vi "run_pharmaBotExp_v0.015.vi"(0 "data in":T12={"daq_ao 1"="Dev1/ao0", "daq_ai 1"="Dev1/ai0", "experiment day folder"=path "C:/multiBot/data/debug/testing", "Multiclamp init error"=0, "Multiclamp Handle Out"=10225184, "sampling rate (Hz)"=20000, "trial name"="t1"}, 1 "auto run?":bool=TRUE, 3 "which manipulator":T13(ring), 4 "HEK/slice options":enum16{"slice", "HEK"}(ring), 5 "error in":errorcluster, 6 "Validate after Experiment":bool, 7 "common cluster":T9, 11 "individual controls in":T8, 13 "images":T3={"slice image"="remote image 000000001461186C", "pipette template"="remote image 000000001461152C", "found pipette"=refnum, "pipette mask for cell tracker"=refnum, "cell images ref"=refnum}) -> (10 "Cell Looks Good?":bool=TRUE, 12 "ValidationOutputCluster":T5(array[cluster]), 14 "ValidationResults":waveform(dbl)[][](array[waveform]), 15 "ValidationPos1":T6(array[ring]), 16 "Exp. Terminated":bool, 17 "ValidationPos2":T6(array[ring]), 18 "ValidationWaveform":waveform(dbl)[](array[waveform]), 19 "error out":errorcluster)   [LabVIEW 2015] (continued)
  in  "Voltage Pulse K":T25={"Which Position to use for Experiment"=enum."Jumper Safe Position", "Duration (s)"=1.0, "Delay (s)"=0.2, "Pulse 2 (s)"=0.4, "Pulse 1 (mV)"=-80.0, "Replicates"=1.0, "Pulse 1 (s)"=0.2, "Pulse 2 (mV)"=-80.0, "Vholding (mV)"=-60.0, "Valve 1 Position"=2, "Valve 2 Position"=2, "Valve 3 Position"=2, "valve 1 used now?"=TRUE, "valve 2 used now?"=FALSE, "valve 3 used now? "=FALSE, "Maintain Final Voltage until end?"=TRUE, "delta Pulse 1 (mV)"=0.0, "delta Pulse 2 (mV)"=5.0, "Sweeps"=24.0, "Final Pulse 1 (mV)"=0.0, "Final Pulse 2 (mV)"=0.0, "protocol Preview"=[]} {"Final Pulse 2 (mV)" step=0.1; "Final Pulse 1 (mV)" step=0.1; "Sweeps" min=1.0 step=1.0; "delta Pulse 2 (mV)" step=0.1; "delta Pulse 1 (mV)" step=0.1; "Valve 3 Position" min=1 max=8; "Valve 2 Position" min=1 max=8; "Valve 1 Position" min=1 max=8; "Vholding (mV)" step=0.1; "Pulse 2 (mV)" step=0.1; "Pulse 1 (s)" min=0.0 step=0.1; "Replicates" min=1.0 step=1.0; "Pulse 1 (mV)" step=0.1; "Pulse 2 (s)" min=0.0 step=0.1; "Delay (s)" min=0.0 step=0.1; "Duration (s)" min=0.0 step=0.1}
  in  "Jump Train K":T26={"Which Position to use for Experiment"=enum."Jumper Safe Position", "Start Position (N)"="", "Jump Position (m)"="", "Duration (s)"=20.0, "Delay (s)"=1.0, "Pulse Width (s)"=1.0, "Valve 1 Position"=1, "Valve 2 Position"=1, "Replicates"=1.0, "Pulse Period (s)"=2.0, "Vholding (mV)"=-60.0, "Number of Pulses"=5.0, "valve 1 used now?"=TRUE, "valve 2 used now?"=FALSE, "valve 3 used now? "=FALSE, "Valve 3 Position"=1, "protocol Preview"=[]} {"Valve 3 Position" min=1 max=8; "Number of Pulses" min=0.0 step=1.0; "Vholding (mV)" step=0.1; "Pulse Period (s)" min=0.0 step=0.1; "Replicates" min=1.0 step=1.0; "Valve 2 Position" min=1 max=8; "Valve 1 Position" min=1 max=8; "Pulse Width (s)" min=0.0 step=0.1; "Delay (s)" min=0.0 step=0.1; "Duration (s)" min=0.0 step=0.1}
  in  "Paired Pulse K":T27={"Which Position to use for Experiment"=enum."Jumper Safe Position", "Start Position (N)"="", "Jump Position (m)"="", "Duration (s)"=10.0, "Delay (s)"=1.0, "Pulse Width (s)"=1.0, "Replicates"=1.0, "Pulse Delay (s)"=1.0, "Pulse Delta Delay (s)"=0.5, "Vholding (mV)"=-60.0, "Valve 1 Position"=1, "Valve 2 Position"=1, "valve 1 used now?"=TRUE, "valve 2 used now?"=FALSE, "valve 3 used now? "=FALSE, "Valve 3 Position"=1, "protocol Preview"=[]} {"Valve 3 Position" min=1 max=8; "Valve 2 Position" min=1 max=8; "Valve 1 Position" min=1 max=8; "Vholding (mV)" step=0.1; "Pulse Delta Delay (s)" min=0.0 step=0.1; "Pulse Delay (s)" min=0.0 step=0.1; "Replicates" min=1.0 step=1.0; "Pulse Width (s)" min=0.0 step=0.1; "Delay (s)" min=0.0 step=0.1; "Duration (s)" min=0.0 step=0.1}
  in  "Single Manip Jump K":T28={"Start Position (N)"=enum."Jumper Position B", "Duration (s)"=8.0, "Delay (s)"=0.5, "Pulse Width (s)"=1.0, "Valve 1 Position"=2, "Valve 2 Position"=2, "Replicates"=10.0, "Jump Position (m)"=enum."Jumper Position A", "Vholding (mV)"=-60.0, "Valve 3 Position"=2, "valve 1 used now?"=TRUE, "valve 2 used now?"=FALSE, "valve 3 used now? "=FALSE, "protocol Preview"=[]} {"Valve 3 Position" min=1 max=8; "Vholding (mV)" step=0.1; "Replicates" min=1.0 step=1.0; "Valve 2 Position" min=1 max=8; "Valve 1 Position" min=1 max=8; "Pulse Width (s)" min=0.0 step=0.1; "Delay (s)" min=0.0 step=0.1; "Duration (s)" min=0.0 step=0.1}
  in  "Gap Free K":T29={"Which Position to use for Experiment"=enum."Jumper Position B", "Duration (s)"=10.0, "Valve 1 Position"=2, "Valve 2 Position"=2, "Replicates"=5.0, "Vholding (mV)"=-60.0, "Valve 3 Position"=2, "valve 1 used now?"=TRUE, "valve 2 used now?"=FALSE, "valve 3 used now? "=FALSE, "Record During Solution Change?"=FALSE} {"Valve 3 Position" min=1 max=8; "Vholding (mV)" step=0.1; "Replicates" min=1.0 step=1.0; "Valve 2 Position" min=1 max=8; "Valve 1 Position" min=1 max=8; "Duration (s)" min=0.0 step=0.1}
  in  "Multi Manip Jump K":T30={"Start Position (N)"=enum."Jumper Position C", "Duration (s)"=20.0, "Delay (s)"=2.0, "Valve 1 Position"=2, "Valve 2 Position"=2, "Replicates"=5.0, "Vholding (mV)"=-60.0, "Valve 3 Position"=2, "valve 1 used now?"=TRUE, "valve 2 used now?"=FALSE, "valve 3 used now? "=FALSE, "Jump Position Array"=[enum."Jumper Position B", enum."Jumper Position A", enum."Jumper Position B", enum."Jumper Position C"], "Position Dwell Time (s)"=[2.0, 4.0, 4.0, 4.0], "protocol Preview"=[]} {"Position Dwell Time (s)" min=0.0 step=0.1; "Vholding (mV)" step=0.1; "Replicates" min=1.0 step=1.0; "Valve 2 Position" min=1 max=8; "Delay (s)" min=0.0 step=0.1; "Duration (s)" min=0.0 step=0.1}
  in  "Current Pulse K":T31={"Which Position to use for Experiment"=enum."Jumper Safe Position", "Duration (s)"=1.0, "Delay (s)"=0.2, "Pulse 2 (s)"=0.4, "Pulse 1 (pA)"=-400.0, "Replicates"=1.0, "Pulse 1 (s)"=0.6, "Pulse 2 (pA)"=-80.0, "Iholding (pA)"=0.0, "Valve 1 Position"=2, "Valve 2 Position"=2, "Valve 3 Position"=2, "valve 1 used now?"=TRUE, "valve 2 used now?"=FALSE, "valve 3 used now? "=FALSE, "Maintain Final Voltage until end?"=FALSE, "delta Pulse 1 (pA)"=50.0, "delta Pulse 2 (pA)"=5.0, "Sweeps"=24.0, "Final Pulse 1 (pA)"=0.0, "Final Pulse 2 (pA)"=0.0, "protocol Preview"=[]} {"Final Pulse 2 (pA)" step=0.1; "Final Pulse 1 (pA)" step=0.1; "Sweeps" min=1.0 step=1.0; "delta Pulse 2 (pA)" step=0.1; "delta Pulse 1 (pA)" step=0.1; "Valve 3 Position" min=1 max=8; "Valve 2 Position" min=1 max=8; "Valve 1 Position" min=1 max=8; "Iholding (pA)" step=0.1; "Pulse 2 (pA)" step=0.1; "Pulse 1 (s)" min=0.0 step=0.1; "Replicates" min=1.0 step=1.0; "Pulse 1 (pA)" step=0.1; "Pulse 2 (s)" min=0.0 step=0.1; "Delay (s)" min=0.0 step=0.1; "Duration (s)" min=0.0 step=0.1}
  in  "Current Ramp K":T32={"Which Position to use for Experiment"=enum."Jumper Safe Position", "Duration (s)"=10.0, "Delay (s)"=1.0, "Ramp Slope (pA/s)"=0.0, "Current Start (pA)"=-200.0, "Replicates"=1.0, "Current End (pA)"=500.0, "Ramp Duration (s)"=5.0, "Iholding (pA)"=0.0, "Valve 1 Position"=2, "Valve 2 Position"=2, "Valve 3 Position"=2, "valve 1 used now?"=TRUE, "valve 2 used now?"=FALSE, "valve 3 used now? "=FALSE, "Maintain Final Voltage until end?"=FALSE, "protocol Preview"=[]} {"Valve 3 Position" min=1 max=8; "Valve 2 Position" min=1 max=8; "Valve 1 Position" min=1 max=8; "Ramp Duration (s)" min=0.0 step=0.1; "Current End (pA)" step=0.1; "Replicates" min=1.0 step=1.0; "Current Start (pA)" step=0.1; "Ramp Slope (pA/s)" step=0.1; "Delay (s)" min=0.0 step=0.1; "Duration (s)" min=0.0 step=0.1}
  in  "Gap Free Iclamp K":T33={"Which Position to use for Experiment"=enum."Don't Move", "Duration (s)"=10.0, "Valve 1 Position"=2, "Valve 2 Position"=2, "Replicates"=5.0, "Iholding (pA)"=200.0, "Valve 3 Position"=2, "valve 1 used now?"=TRUE, "valve 2 used now?"=FALSE, "valve 3 used now? "=FALSE, "Record During Solution Change?"=FALSE} {"Valve 3 Position" min=1 max=8; "Iholding (pA)" step=0.1; "Replicates" min=1.0 step=1.0; "Valve 2 Position" min=1 max=8; "Valve 1 Position" min=1 max=8; "Duration (s)" min=0.0 step=0.1}
  in  "PhaseL Experiment Option":string(combo)="Single Manip Jump"
  in  "Experiment Selection L":T20(tab)=enum."Paired Pulse"
  in  "Single Jump L":T21={"Which Position to use for Experiment"=enum."Jumper Position B-A", "Start Position (N)"="Jumper Posistion B", "Jump Position (m)"="Jumper Posistion A", "Duration (s)"=5.0, "Delay (s)"=1.0, "Pulse Width (s)"=1.0, "Valve 1 Position"=2, "Valve 2 Position"=2, "Replicates"=10.0, "Vholding (mV)"=-60.0, "Valve 3 Position"=2, "valve 1 used now?"=TRUE, "valve 2 used now?"=FALSE, "valve 3 used now? "=FALSE, "protocol Preview"=[]} {"Valve 3 Position" min=1 max=8; "Vholding (mV)" step=0.1; "Replicates" min=1.0 step=1.0; "Valve 2 Position" min=1 max=8; "Valve 1 Position" min=1 max=8; "Pulse Width (s)" min=0.0 step=0.1; "Delay (s)" min=0.0 step=0.1; "Duration (s)" min=0.0 step=0.1}
  in  "Solution Change L":T22={"Which Position to use for Experiment"=enum."Jumper Safe Position", "Duration (s)"=60.0, "Delay (s)"=1.0, "Pulse Width (s)"=30.0, "Which Valve to Change?"=1, "Valve Jump Position"=3, "Replicates"=1.0, "Vholding (mV)"=-70.0, "valve 1 used now?"=TRUE, "valve 2 used now?"=FALSE, "valve 3 used now? "=FALSE, "Valve 1 Position"=2, "Valve 2 Position"=2, "Valve 3 Position"=2, "protocol Preview"=[]} {"Valve 3 Position" min=1 max=8; "Valve 2 Position" min=1 max=8; "Valve 1 Position" min=1 max=8; "Vholding (mV)" step=0.1; "Replicates" min=1.0 step=1.0; "Valve Jump Position" min=1 max=8 step=1; "Which Valve to Change?" min=1 max=8 step=1; "Pulse Width (s)" min=0.0 step=0.1; "Delay (s)" min=0.0 step=0.1; "Duration (s)" min=0.0 step=0.1}
  in  "Voltage Step L":T23={"Which Position to use for Experiment"=enum."Jumper Safe Position", "Duration (s)"=10.0, "Delay (s)"=1.0, "Step Width (s)"=0.1, "Voltage Start (mV)"=-60.0, "Voltage Step (mV)"=0.0, "Replicates"=1.0, "Voltage End (mV)"=40.0, "Number of Step"=20.0, "Vholding (mV)"=-60.0, "Valve 1 Position"=2, "Valve 2 Position"=2, "Valve 3 Position"=2, "valve 1 used now?"=TRUE, "valve 2 used now?"=FALSE, "valve 3 used now? "=FALSE, "Total Step Time (s)"=0.0, "Maintain Final Voltage until end?"=TRUE, "protocol Preview"=[]} {"Total Step Time (s)" min=0.0 step=0.1; "Valve 3 Position" min=1 max=8; "Valve 2 Position" min=1 max=8; "Valve 1 Position" min=1 max=8; "Vholding (mV)" step=0.1; "Number of Step" min=0.0 step=1.0; "Voltage End (mV)" step=0.1; "Replicates" min=1.0 step=1.0; "Voltage Step (mV)" step=0.1; "Voltage Start (mV)" step=0.1; "Step Width (s)" step=0.1; "Delay (s)" min=0.0 step=0.1; "Duration (s)" min=0.0 step=0.1}
  in  "Voltage Ramp L":T24={"Which Position to use for Experiment"=enum."Jumper Safe Position", "Duration (s)"=10.0, "Delay (s)"=1.0, "Ramp Slope (mV/s)"=0.0, "Voltage Start (mV)"=-60.0, "Replicates"=1.0, "Voltage End (mV)"=40.0, "Ramp Duration (s)"=5.0, "Vholding (mV)"=-60.0, "Valve 1 Position"=2, "Valve 2 Position"=2, "Valve 3 Position"=2, "valve 1 used now?"=TRUE, "valve 2 used now?"=FALSE, "valve 3 used now? "=FALSE, "Maintain Final Voltage until end?"=TRUE, "protocol Preview"=[]} {"Valve 3 Position" min=1 max=8; "Valve 2 Position" min=1 max=8; "Valve 1 Position" min=1 max=8; "Ramp Duration (s)" min=0.0 step=0.1; "Voltage End (mV)" step=0.1; "Replicates" min=1.0 step=1.0; "Voltage Start (mV)" step=0.1; "Ramp Slope (mV/s)" step=0.1; "Delay (s)" min=0.0 step=0.1; "Duration (s)" min=0.0 step=0.1}
  in  "Voltage Pulse L":T25={"Which Position to use for Experiment"=enum."Jumper Safe Position", "Duration (s)"=1.0, "Delay (s)"=0.2, "Pulse 2 (s)"=0.4, "Pulse 1 (mV)"=-80.0, "Replicates"=1.0, "Pulse 1 (s)"=0.2, "Pulse 2 (mV)"=-80.0, "Vholding (mV)"=-60.0, "Valve 1 Position"=2, "Valve 2 Position"=2, "Valve 3 Position"=2, "valve 1 used now?"=TRUE, "valve 2 used now?"=FALSE, "valve 3 used now? "=FALSE, "Maintain Final Voltage until end?"=TRUE, "delta Pulse 1 (mV)"=0.0, "delta Pulse 2 (mV)"=5.0, "Sweeps"=24.0, "Final Pulse 1 (mV)"=0.0, "Final Pulse 2 (mV)"=0.0, "protocol Preview"=[]} {"Final Pulse 2 (mV)" step=0.1; "Final Pulse 1 (mV)" step=0.1; "Sweeps" min=1.0 step=1.0; "delta Pulse 2 (mV)" step=0.1; "delta Pulse 1 (mV)" step=0.1; "Valve 3 Position" min=1 max=8; "Valve 2 Position" min=1 max=8; "Valve 1 Position" min=1 max=8; "Vholding (mV)" step=0.1; "Pulse 2 (mV)" step=0.1; "Pulse 1 (s)" min=0.0 step=0.1; "Replicates" min=1.0 step=1.0; "Pulse 1 (mV)" step=0.1; "Pulse 2 (s)" min=0.0 step=0.1; "Delay (s)" min=0.0 step=0.1; "Duration (s)" min=0.0 step=0.1}
  in  "Jump Train L":T26={"Which Position to use for Experiment"=enum."Jumper Safe Position", "Start Position (N)"="", "Jump Position (m)"="", "Duration (s)"=20.0, "Delay (s)"=1.0, "Pulse Width (s)"=1.0, "Valve 1 Position"=1, "Valve 2 Position"=1, "Replicates"=1.0, "Pulse Period (s)"=2.0, "Vholding (mV)"=-60.0, "Number of Pulses"=5.0, "valve 1 used now?"=TRUE, "valve 2 used now?"=FALSE, "valve 3 used now? "=FALSE, "Valve 3 Position"=1, "protocol Preview"=[]} {"Valve 3 Position" min=1 max=8; "Number of Pulses" min=0.0 step=1.0; "Vholding (mV)" step=0.1; "Pulse Period (s)" min=0.0 step=0.1; "Replicates" min=1.0 step=1.0; "Valve 2 Position" min=1 max=8; "Valve 1 Position" min=1 max=8; "Pulse Width (s)" min=0.0 step=0.1; "Delay (s)" min=0.0 step=0.1; "Duration (s)" min=0.0 step=0.1}
  in  "Paired Pulse L":T27={"Which Position to use for Experiment"=enum."Jumper Safe Position", "Start Position (N)"="", "Jump Position (m)"="", "Duration (s)"=10.0, "Delay (s)"=1.0, "Pulse Width (s)"=1.0, "Replicates"=1.0, "Pulse Delay (s)"=1.0, "Pulse Delta Delay (s)"=0.5, "Vholding (mV)"=-60.0, "Valve 1 Position"=1, "Valve 2 Position"=1, "valve 1 used now?"=TRUE, "valve 2 used now?"=FALSE, "valve 3 used now? "=FALSE, "Valve 3 Position"=1, "protocol Preview"=[]} {"Valve 3 Position" min=1 max=8; "Valve 2 Position" min=1 max=8; "Valve 1 Position" min=1 max=8; "Vholding (mV)" step=0.1; "Pulse Delta Delay (s)" min=0.0 step=0.1; "Pulse Delay (s)" min=0.0 step=0.1; "Replicates" min=1.0 step=1.0; "Pulse Width (s)" min=0.0 step=0.1; "Delay (s)" min=0.0 step=0.1; "Duration (s)" min=0.0 step=0.1}
  in  "Single Manip Jump L":T28={"Start Position (N)"=enum."Jumper Position B", "Duration (s)"=8.0, "Delay (s)"=0.5, "Pulse Width (s)"=1.0, "Valve 1 Position"=2, "Valve 2 Position"=2, "Replicates"=10.0, "Jump Position (m)"=enum."Jumper Position A", "Vholding (mV)"=-60.0, "Valve 3 Position"=2, "valve 1 used now?"=TRUE, "valve 2 used now?"=FALSE, "valve 3 used now? "=FALSE, "protocol Preview"=[]} {"Valve 3 Position" min=1 max=8; "Vholding (mV)" step=0.1; "Replicates" min=1.0 step=1.0; "Valve 2 Position" min=1 max=8; "Valve 1 Position" min=1 max=8; "Pulse Width (s)" min=0.0 step=0.1; "Delay (s)" min=0.0 step=0.1; "Duration (s)" min=0.0 step=0.1}
  in  "Gap Free L":T29={"Which Position to use for Experiment"=enum."Jumper Position B", "Duration (s)"=10.0, "Valve 1 Position"=2, "Valve 2 Position"=2, "Replicates"=5.0, "Vholding (mV)"=-60.0, "Valve 3 Position"=2, "valve 1 used now?"=TRUE, "valve 2 used now?"=FALSE, "valve 3 used now? "=FALSE, "Record During Solution Change?"=FALSE} {"Valve 3 Position" min=1 max=8; "Vholding (mV)" step=0.1; "Replicates" min=1.0 step=1.0; "Valve 2 Position" min=1 max=8; "Valve 1 Position" min=1 max=8; "Duration (s)" min=0.0 step=0.1}
  in  "Multi Manip Jump L":T30={"Start Position (N)"=enum."Jumper Position C", "Duration (s)"=20.0, "Delay (s)"=2.0, "Valve 1 Position"=2, "Valve 2 Position"=2, "Replicates"=5.0, "Vholding (mV)"=-60.0, "Valve 3 Position"=2, "valve 1 used now?"=TRUE, "valve 2 used now?"=FALSE, "valve 3 used now? "=FALSE, "Jump Position Array"=[enum."Jumper Position B", enum."Jumper Position A", enum."Jumper Position B", enum."Jumper Position C"], "Position Dwell Time (s)"=[2.0, 4.0, 4.0, 4.0], "protocol Preview"=[]} {"Position Dwell Time (s)" min=0.0 step=0.1; "Vholding (mV)" step=0.1; "Replicates" min=1.0 step=1.0; "Valve 2 Position" min=1 max=8; "Delay (s)" min=0.0 step=0.1; "Duration (s)" min=0.0 step=0.1}
  in  "Current Pulse L":T31={"Which Position to use for Experiment"=enum."Jumper Safe Position", "Duration (s)"=1.0, "Delay (s)"=0.2, "Pulse 2 (s)"=0.4, "Pulse 1 (pA)"=-400.0, "Replicates"=1.0, "Pulse 1 (s)"=0.6, "Pulse 2 (pA)"=-80.0, "Iholding (pA)"=0.0, "Valve 1 Position"=2, "Valve 2 Position"=2, "Valve 3 Position"=2, "valve 1 used now?"=TRUE, "valve 2 used now?"=FALSE, "valve 3 used now? "=FALSE, "Maintain Final Voltage until end?"=FALSE, "delta Pulse 1 (pA)"=50.0, "delta Pulse 2 (pA)"=5.0, "Sweeps"=24.0, "Final Pulse 1 (pA)"=0.0, "Final Pulse 2 (pA)"=0.0, "protocol Preview"=[]} {"Final Pulse 2 (pA)" step=0.1; "Final Pulse 1 (pA)" step=0.1; "Sweeps" min=1.0 step=1.0; "delta Pulse 2 (pA)" step=0.1; "delta Pulse 1 (pA)" step=0.1; "Valve 3 Position" min=1 max=8; "Valve 2 Position" min=1 max=8; "Valve 1 Position" min=1 max=8; "Iholding (pA)" step=0.1; "Pulse 2 (pA)" step=0.1; "Pulse 1 (s)" min=0.0 step=0.1; "Replicates" min=1.0 step=1.0; "Pulse 1 (pA)" step=0.1; "Pulse 2 (s)" min=0.0 step=0.1; "Delay (s)" min=0.0 step=0.1; "Duration (s)" min=0.0 step=0.1}
  in  "Current Ramp L":T32={"Which Position to use for Experiment"=enum."Jumper Safe Position", "Duration (s)"=10.0, "Delay (s)"=1.0, "Ramp Slope (pA/s)"=0.0, "Current Start (pA)"=-200.0, "Replicates"=1.0, "Current End (pA)"=500.0, "Ramp Duration (s)"=5.0, "Iholding (pA)"=0.0, "Valve 1 Position"=2, "Valve 2 Position"=2, "Valve 3 Position"=2, "valve 1 used now?"=TRUE, "valve 2 used now?"=FALSE, "valve 3 used now? "=FALSE, "Maintain Final Voltage until end?"=FALSE, "protocol Preview"=[]} {"Valve 3 Position" min=1 max=8; "Valve 2 Position" min=1 max=8; "Valve 1 Position" min=1 max=8; "Ramp Duration (s)" min=0.0 step=0.1; "Current End (pA)" step=0.1; "Replicates" min=1.0 step=1.0; "Current Start (pA)" step=0.1; "Ramp Slope (pA/s)" step=0.1; "Delay (s)" min=0.0 step=0.1; "Duration (s)" min=0.0 step=0.1}
  in  "Gap Free Iclamp L":T33={"Which Position to use for Experiment"=enum."Don't Move", "Duration (s)"=10.0, "Valve 1 Position"=2, "Valve 2 Position"=2, "Replicates"=5.0, "Iholding (pA)"=200.0, "Valve 3 Position"=2, "valve 1 used now?"=TRUE, "valve 2 used now?"=FALSE, "valve 3 used now? "=FALSE, "Record During Solution Change?"=FALSE} {"Valve 3 Position" min=1 max=8; "Iholding (pA)" step=0.1; "Replicates" min=1.0 step=1.0; "Valve 2 Position" min=1 max=8; "Valve 1 Position" min=1 max=8; "Duration (s)" min=0.0 step=0.1}
  in  "ending set":enum32{"Iprot", "Vprot", "Imemtest", "Vmemtest"}(tab)
  in  "holding memtest":bool=TRUE
  in  "holding set":enum32{"VClamp", "IClamp"}(tab)
  out "holding vmemtest cmd":waveform(dbl)(graph)
  in  "holding Vclamp memtest":T17={"Samples to Read"=2000, "Rate (Hz)"=20000.0, "Amplitude (mV/pA)"=10.0, "Offset (mV/pA)"=0.0, "Frequency (Hz)"=10.0, "duty cycle (%)"=50.0, "phase"=-90.0} {"phase" format="%.2p"; "duty cycle (%)" format="%0.2f"}
  out "holding imemtest cmd":waveform(dbl)(graph)
  in  "holding Iclamp memtest":T17={"Samples to Read"=2000, "Rate (Hz)"=20000.0, "Amplitude (mV/pA)"=-50.0, "Offset (mV/pA)"=0.0, "Frequency (Hz)"=10.0, "duty cycle (%)"=50.0, "phase"=0.0} {"phase" format="%.2p"; "duty cycle (%)" format="%0.2f"}
  # "(will skip all subsequent Phases)"
  # "Checks Twitter for user Control\npharmaBotEmory\nga12345"
  # "IClamp step protocol"
  # "x"
  # "VClamp step protocol"
  # "x"
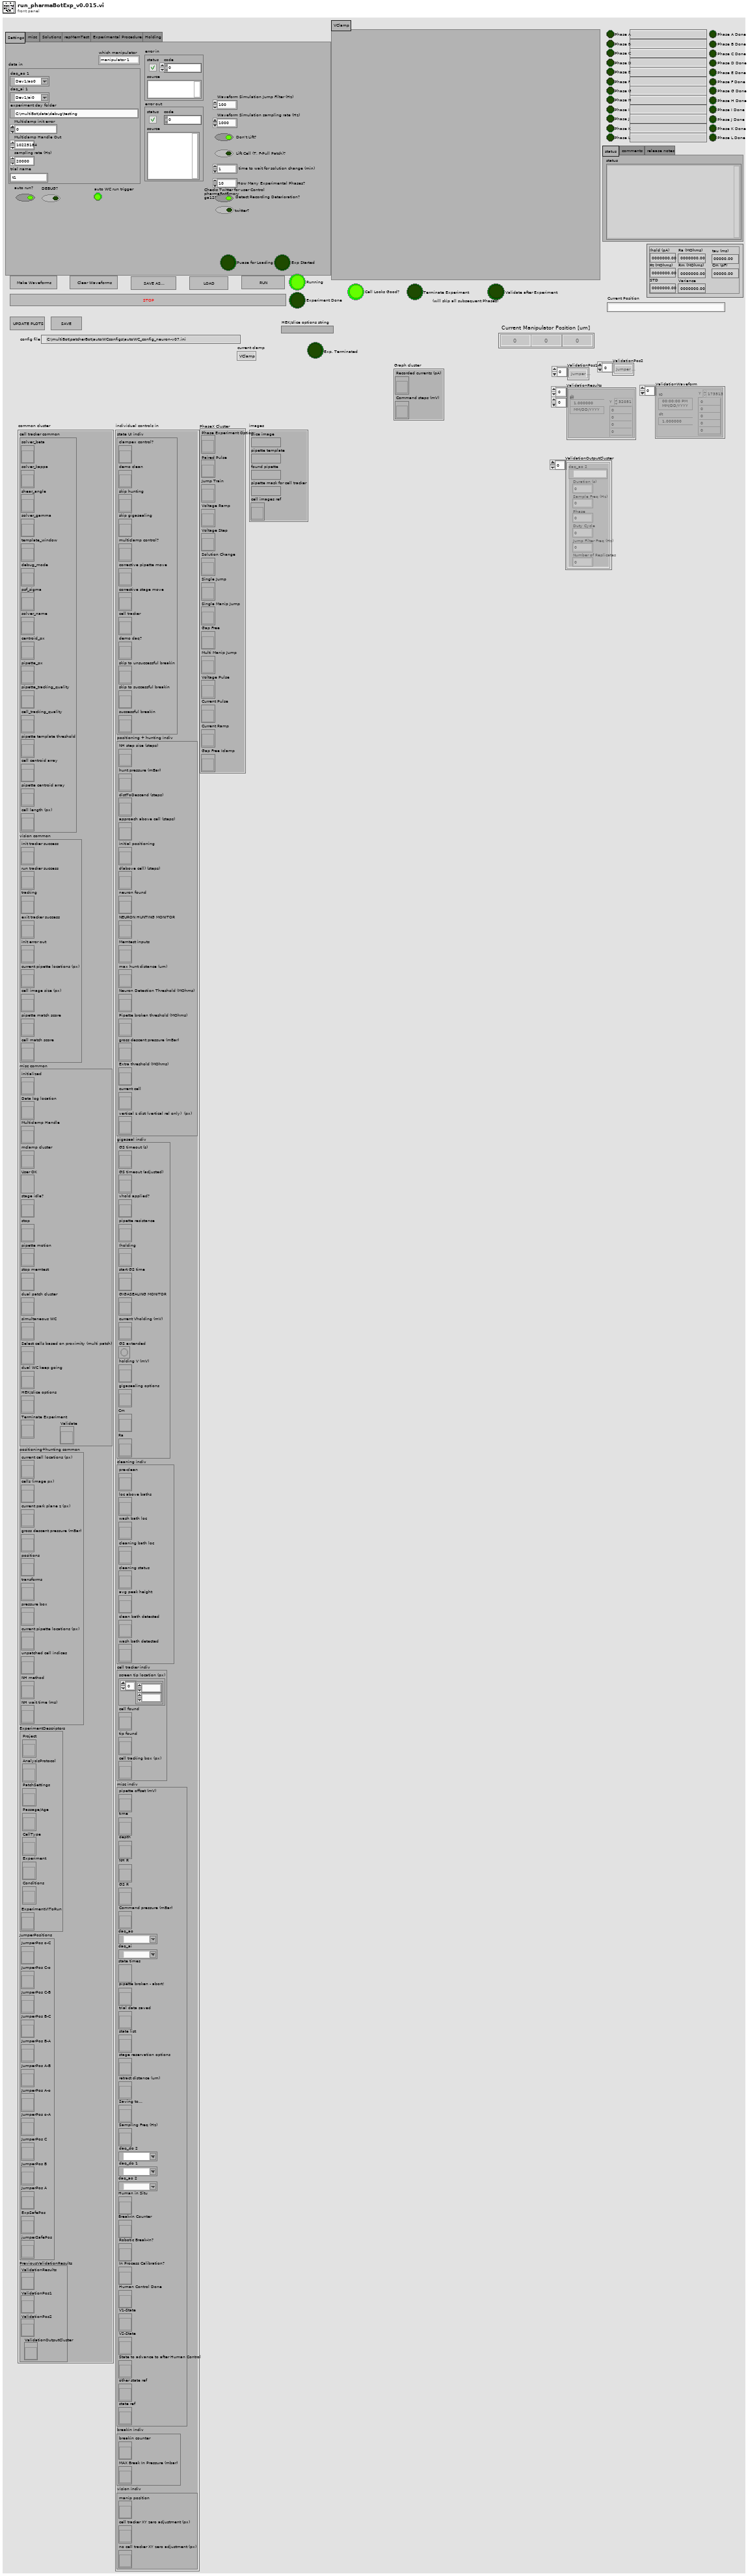
[diagram p1: front panel]
types:
  T1 = cluster{"Phase Experiment Option":refnum<vi>, "Paired Pulse":refnum<vi>, "Jump Train":refnum<vi>, "Voltage Ramp":refnum<vi>, "Voltage Step":refnum<vi>, "Solution Change":refnum<vi>, "Single Jump":refnum<vi>, "Single Manip Jump":refnum<vi>, "Gap Free":refnum<vi>, "Multi Manip Jump":refnum<vi>, "Voltage Pulse":refnum<vi>, "Current Pulse":refnum<vi>, "Current Ramp":refnum<vi>, "Gap Free Iclamp":refnum<vi>}
  T2 = cluster{"How Many Experimental Phases?":refnum<vi>, "PhaseA Cluster":cluster{"Phase Experiment Option":refnum<vi>, "Paired Pulse":refnum<vi>, "Jump Train":refnum<vi>, "Voltage Ramp":refnum<vi>, "Voltage Step":refnum<vi>, "Solution Change":refnum<vi>, "Single Jump":refnum<vi>, "Single Manip Jump":refnum<vi>, "Gap Free":refnum<vi>, "Multi Manip Jump":refnum<vi>, "Voltage Pulse":refnum<vi>, "Current Pulse":refnum<vi>, "Current Ramp":refnum<vi>, "Gap Free Iclamp":refnum<vi>}, "PhaseB Cluster":cluster{"Phase Experiment Option":refnum<vi>, "Paired Pulse":refnum<vi>, "Jump Train":refnum<vi>, "Voltage Ramp":refnum<vi>, "Voltage Step":refnum<vi>, "Solution Change":refnum<vi>, "Single Jump":refnum<vi>, "Single Manip Jump":refnum<vi>, "Gap Free":refnum<vi>, "Multi Manip Jump":refnum<vi>, "Voltage Pulse":refnum<vi>, "Current Pulse":refnum<vi>, "Current Ramp":refnum<vi>, "Gap Free Iclamp":refnum<vi>}, "PhaseC Cluster":cluster{"Phase Experiment Option":refnum<vi>, "Paired Pulse":refnum<vi>, "Jump Train":refnum<vi>, "Voltage Ramp":refnum<vi>, "Voltage Step":refnum<vi>, "Solution Change":refnum<vi>, "Single Jump":refnum<vi>, "Single Manip Jump":refnum<vi>, "Gap Free":refnum<vi>, "Multi Manip Jump":refnum<vi>, "Voltage Pulse":refnum<vi>, "Current Pulse":refnum<vi>, "Current Ramp":refnum<vi>, "Gap Free Iclamp":refnum<vi>}, "PhaseD Cluster":cluster{"Phase Experiment Option":refnum<vi>, "Paired Pulse":refnum<vi>, "Jump Train":refnum<vi>, "Voltage Ramp":refnum<vi>, "Voltage Step":refnum<vi>, "Solution Change":refnum<vi>, "Single Jump":refnum<vi>, "Single Manip Jump":refnum<vi>, "Gap Free":refnum<vi>, "Multi Manip Jump":refnum<vi>, "Voltage Pulse":refnum<vi>, "Current Pulse":refnum<vi>, "Current Ramp":refnum<vi>, "Gap Free Iclamp":refnum<vi>}, "PhaseE Cluster":cluster{"Phase Experiment Option":refnum<vi>, "Paired Pulse":refnum<vi>, "Jump Train":refnum<vi>, "Voltage Ramp":refnum<vi>, "Voltage Step":refnum<vi>, "Solution Change":refnum<vi>, "Single Jump":refnum<vi>, "Single Manip Jump":refnum<vi>, "Gap Free":refnum<vi>, "Multi Manip Jump":refnum<vi>, "Voltage Pulse":refnum<vi>, "Current Pulse":refnum<vi>, "Current Ramp":refnum<vi>, "Gap Free Iclamp":refnum<vi>}, "PhaseF Cluster":cluster{"Phase Experiment Option":refnum<vi>, "Paired Pulse":refnum<vi>, "Jump Train":refnum<vi>, "Voltage Ramp":refnum<vi>, "Voltage Step":refnum<vi>, "Solution Change":refnum<vi>, "Single Jump":refnum<vi>, "Single Manip Jump":refnum<vi>, "Gap Free":refnum<vi>, "Multi Manip Jump":refnum<vi>, "Voltage Pulse":refnum<vi>, "Current Pulse":refnum<vi>, "Current Ramp":refnum<vi>, "Gap Free Iclamp":refnum<vi>}, "time to wait for solution change (min)":refnum<vi>, "valve Time Cluster":cluster{"time of Last V1 Change":refnum<vi>, "time of Last V2 Change":refnum<vi>, "time of Last V3 Change":refnum<vi>}, "PhaseG Cluster":cluster{"Phase Experiment Option":refnum<vi>, "Paired Pulse":refnum<vi>, "Jump Train":refnum<vi>, "Voltage Ramp":refnum<vi>, "Voltage Step":refnum<vi>, "Solution Change":refnum<vi>, "Single Jump":refnum<vi>, "Single Manip Jump":refnum<vi>, "Gap Free":refnum<vi>, "Multi Manip Jump":refnum<vi>, "Voltage Pulse":refnum<vi>, "Current Pulse":refnum<vi>, "Current Ramp":refnum<vi>, "Gap Free Iclamp":refnum<vi>}, "PhaseH Cluster":cluster{"Phase Experiment Option":refnum<vi>, "Paired Pulse":refnum<vi>, "Jump Train":refnum<vi>, "Voltage Ramp":refnum<vi>, "Voltage Step":refnum<vi>, "Solution Change":refnum<vi>, "Single Jump":refnum<vi>, "Single Manip Jump":refnum<vi>, "Gap Free":refnum<vi>, "Multi Manip Jump":refnum<vi>, "Voltage Pulse":refnum<vi>, "Current Pulse":refnum<vi>, "Current Ramp":refnum<vi>, "Gap Free Iclamp":refnum<vi>}, "PhaseI Cluster":cluster{"Phase Experiment Option":refnum<vi>, "Paired Pulse":refnum<vi>, "Jump Train":refnum<vi>, "Voltage Ramp":refnum<vi>, "Voltage Step":refnum<vi>, "Solution Change":refnum<vi>, "Single Jump":refnum<vi>, "Single Manip Jump":refnum<vi>, "Gap Free":refnum<vi>, "Multi Manip Jump":refnum<vi>, "Voltage Pulse":refnum<vi>, "Current Pulse":refnum<vi>, "Current Ramp":refnum<vi>, "Gap Free Iclamp":refnum<vi>}, "PhaseJ Cluster":cluster{"Phase Experiment Option":refnum<vi>, "Paired Pulse":refnum<vi>, "Jump Train":refnum<vi>, "Voltage Ramp":refnum<vi>, "Voltage Step":refnum<vi>, "Solution Change":refnum<vi>, "Single Jump":refnum<vi>, "Single Manip Jump":refnum<vi>, "Gap Free":refnum<vi>, "Multi Manip Jump":refnum<vi>, "Voltage Pulse":refnum<vi>, "Current Pulse":refnum<vi>, "Current Ramp":refnum<vi>, "Gap Free Iclamp":refnum<vi>}, "PhaseK Cluster":cluster{"Phase Experiment Option":refnum<vi>, "Paired Pulse":refnum<vi>, "Jump Train":refnum<vi>, "Voltage Ramp":refnum<vi>, "Voltage Step":refnum<vi>, "Solution Change":refnum<vi>, "Single Jump":refnum<vi>, "Single Manip Jump":refnum<vi>, "Gap Free":refnum<vi>, "Multi Manip Jump":refnum<vi>, "Voltage Pulse":refnum<vi>, "Current Pulse":refnum<vi>, "Current Ramp":refnum<vi>, "Gap Free Iclamp":refnum<vi>}, "PhaseL Cluster":cluster{"Phase Experiment Option":refnum<vi>, "Paired Pulse":refnum<vi>, "Jump Train":refnum<vi>, "Voltage Ramp":refnum<vi>, "Voltage Step":refnum<vi>, "Solution Change":refnum<vi>, "Single Jump":refnum<vi>, "Single Manip Jump":refnum<vi>, "Gap Free":refnum<vi>, "Multi Manip Jump":refnum<vi>, "Voltage Pulse":refnum<vi>, "Current Pulse":refnum<vi>, "Current Ramp":refnum<vi>, "Gap Free Iclamp":refnum<vi>}, "PhaseStatusCluster":cluster{"Phase A Done":refnum<vi>, "Phase B Done":refnum<vi>, "Phase C Done":refnum<vi>, "Phase D Done":refnum<vi>, "Phase E Done":refnum<vi>, "Phase F Done":refnum<vi>, "Phase G Done":refnum<vi>, "Phase H Done":refnum<vi>, "Phase I Done":refnum<vi>, "Phase J Done":refnum<vi>, "Phase K Done":refnum<vi>, "Phase L Done":refnum<vi>}}
  T3 = typedef "images_controls.ctl" = cluster{"slice image":T4, "pipette template":T4, "found pipette":T4, "pipette mask for cell tracker":T4, "cell images ref":refnum<vi>}
  T4 = typedef "IMAQ Image.ctl" = refnum<image>
  T5 = cluster{"daq_ao 2":tag, "Duration (s)":dbl, "Sample Freq (Hz)":dbl, "Phase":dbl, "Duty Cycle":dbl, "Jump Filter Freq (Hz)":dbl, "Number of Replicates":i16}[]
  T6 = enum16{"Jumper Safe Position", "Experiment Safe Position", "Jumper Position A", "Jumper Position B", "Jumper Position C", "Jumper Position o-A", "Jumper Position A-o", "Jumper Position A-B", "Jumper Position B-A", "Jumper Position B-C", "Jumper Position C-B", "Jumper Position C-o", "Jumper Position o-C"}[]
  T7 = cluster{"Recorded currents (pA)":refnum<vi>, "Command steps (mV)":refnum<vi>}
  T8 = typedef "multipatch_individual_controls_v5.ctl" = cluster{"state UI indiv":cluster{"clampex control?":refnum<vi>, "demo clean":refnum<vi>, "skip hunting":refnum<vi>, "skip gigasealing":refnum<vi>, "multiclamp control?":refnum<vi>, "corrective pipette move":refnum<vi>, "corrective stage move":refnum<vi>, "cell tracker":refnum<vi>, "demo daq?":refnum<vi>, "skip to unsuccessful breakin":refnum<vi>, "skip to successful breakin":refnum<vi>, "successful breakin":refnum<vi>}, "positioning + hunting indiv":cluster{"NH step size (steps)":refnum<vi>, "hunt pressure (mBar)":refnum<vi>, "distToDescend (steps)":refnum<vi>, "approach above cell (steps)":refnum<vi>, "initial positioning":refnum<vi>, "d(above cell) (steps)":refnum<vi>, "neuron found":refnum<vi>, "NEURON HUNTING MONITOR":refnum<vi>, "Memtest inputs":refnum<vi>, "max hunt distance (um)":refnum<vi>, "Neuron Detection Threshold (MOhms)":refnum<vi>, "Pipette broken threshold (MOhms)":refnum<vi>, "gross descent pressure (mBar)":refnum<vi>, "Extra threshold (MOhms)":refnum<vi>, "current cell":refnum<vi>, "vertical z dist (vertical rel only)  (px)":refnum<vi>}, "gigaseal indiv":cluster{"GS timeout (s)":refnum<vi>, "GS timeout (adjusted)":refnum<vi>, "vhold applied?":refnum<vi>, "pipette resistance":refnum<vi>, "Iholding":refnum<vi>, "start GS time":refnum<vi>, "GIGASEALING MONITOR":refnum<vi>, "current Vholding (mV)":refnum<vi>, "GS extended":refnum<vi>, "holding V (mV)":refnum<vi>, "gigasealing options":refnum<vi>, "Cm":refnum<vi>, "Ra ":refnum<vi>}, "cleaning indiv":cluster{"pre-clean":refnum<vi>, "loc above baths":refnum<vi>, "wash bath loc":refnum<vi>, "cleaning bath loc":refnum<vi>, "cleaning status":refnum<vi>, "avg peak height":refnum<vi>, "clean bath detected":refnum<vi>, "wash bath detected":refnum<vi>}, "cell tracker indiv":cluster{"screen tip location (px)":refnum<vi>, "cell found":refnum<vi>, "tip found":refnum<vi>, "cell tracking box (px)":refnum<vi>}, "misc indiv":cluster{"pipette offset (mV)":refnum<vi>, "time":refnum<vi>, "depth":refnum<vi>, "NH R":refnum<vi>, "GS R":refnum<vi>, "Command pressure (mBar)":refnum<vi>, "daq_ao":tag, "daq_ai":tag, "state times":refnum<vi>, "pipette broken - abort!":refnum<vi>, "trial data saved":refnum<vi>, "state list":refnum<vi>, "stage reservation options":refnum<vi>, "retract distance (um)":refnum<vi>, "Saving to...":refnum<vi>, "Sampling Freq (Hz)":refnum<vi>, "daq_do 2":tag, "daq_do 1":tag, "daq_ao 2":tag, "Human in Situ":refnum<vi>, "Break-In Counter":refnum<vi>, "Robotic Break-In?":refnum<vi>, "In Process Calibration?":refnum<vi>, "Human Control Done":refnum<vi>, "V1-State":refnum<vi>, "V2-State":refnum<vi>, "State to advance to after Human Control":refnum<vi>, "other state ref":refnum<vi>, "state ref":refnum<vi>}, "breakin indiv":cluster{"breakin counter":refnum<vi>, "MAX Break In Pressure (mbar)":refnum<vi>}, "vision indiv":cluster{"manip position":refnum<vi>, "cell tracker XY zero adjustment (px)":refnum<vi>, "no cell tracker XY zero adjustment (px)":refnum<vi>}}
  T9 = typedef "multipatch_common_controls_v4.ctl" = cluster{"cell tracker common":cluster{"solver_beta":refnum<vi>, "solver_kappa":refnum<vi>, "shear_angle":refnum<vi>, "solver_gamma":refnum<vi>, "template_window":refnum<vi>, "debug_mode":refnum<vi>, "psf_sigma":refnum<vi>, "solver_name":refnum<vi>, "centroid_px":refnum<vi>, "pipette_px":refnum<vi>, "pipette_tracking_quality":refnum<vi>, "cell_tracking_quality":refnum<vi>, "pipette template threshold":refnum<vi>, "cell centroid array":refnum<vi>, "pipette centroid array":refnum<vi>, "cell length (px)":refnum<vi>}, "vision common":cluster{"init tracker success":refnum<vi>, "run tracker success":refnum<vi>, "tracking":refnum<vi>, "exit tracker success":refnum<vi>, "init error out":refnum<vi>, "current pipette locations (px)":refnum<vi>, "cell image size (px)":refnum<vi>, "pipette match score":refnum<vi>, "cell match score":refnum<vi>}, "misc common":cluster{"initialized":refnum<vi>, "Data log location":refnum<vi>, "Multiclamp Handle":refnum<vi>, "mclamp cluster":refnum<vi>, "User OK":refnum<vi>, "stage idle?":refnum<vi>, "stop":refnum<vi>, "pipette motion":refnum<vi>, "stop memtest":refnum<vi>, "dual patch cluster":refnum<vi>, "simultaneous WC":refnum<vi>, "Select cells based on proximity (multi patch)":refnum<vi>, "dual WC keep going":refnum<vi>, "HEK/slice options":refnum<vi>, "Terminate Experiment":refnum<vi>, "Validate":refnum<vi>}, "positioning+hunting common":cluster{"current cell locations (px)":refnum<vi>, "cells (image px)":refnum<vi>, "current park plane z (px)":refnum<vi>, "gross descent pressure (mBar)":refnum<vi>, "positions":refnum<vi>, "transforms":refnum<vi>, "pressure box":refnum<vi>, "current pipette locations (px)":refnum<vi>, "unpatched cell indices":refnum<vi>, "NH method":refnum<vi>, "NH wait time (ms)":refnum<vi>}, "ExperimentDescriptors":cluster{"Project":refnum<vi>, "AnalysisProtocol":refnum<vi>, "PatchSettings":refnum<vi>, "Passage/Age":refnum<vi>, "CellType":refnum<vi>, "Experiment":refnum<vi>, "Conditions":refnum<vi>, "ExperimentVIToRun":refnum<vi>}, "JumperPositions":cluster{"JumperPos o-C":refnum<vi>, "JumperPos C-o":refnum<vi>, "JumperPos C-B":refnum<vi>, "JumperPos B-C":refnum<vi>, "JumperPos B-A":refnum<vi>, "JumperPos A-B":refnum<vi>, "JumperPos A-o":refnum<vi>, "JumperPos o-A":refnum<vi>, "JumperPos C":refnum<vi>, "JumperPos B":refnum<vi>, "JumperPos A":refnum<vi>, "ExpSafePos":refnum<vi>, "jumperSafePos":refnum<vi>}, "PreviousValidationResults":cluster{"ValidationResults":refnum<vi>, "ValidationPos1":refnum<vi>, "ValidationPos2":refnum<vi>, "ValidationOutputCluster":refnum<vi>}}
  T10 = typedef "cell_stats-v02.ctl" = cluster{"Ihold (pA)":dbl, "Rm (MOhms)":dbl, "Ra (MOhms)":dbl, "Cm (pF)":dbl, "tau (ms)":dbl, "Rt (MOhms)":dbl, "Variance":dbl, "STD":dbl}
  T11 = enum32{"Settings", "misc", "Solutions", "repMemTest", "Experimental Procedures", "Validation", "Holding"}
  T12 = typedef "Data.ctl" = cluster{"daq_ao 1":tag, "daq_ai 1":tag, "experiment day folder":path, "Multiclamp init error":i32, "Multiclamp Handle Out":u32, "sampling rate (Hz)":i32, "trial name":string}
  T13 = enum16{"manipulator 1", "manipulator 2", "manipulator 3", "manipulator 4"}
  T14 = typedef "clamp_profile.ctl" = cluster{"aLevel":dbl, "aDelta":dbl, "aDuration":i32, "bLevel":dbl, "bDelta":dbl, "bDuration":i32, "cLevel":dbl, "cDelta":dbl, "cDuration":i32}
  T15 = cluster{"Iclamp in":T14, "# iter":i32, "# reps IC":i32}
  T16 = cluster{"Vclamp in":T14, "# iter":i32, "# reps VC":i32}
  T17 = typedef "memtest_def.ctl" = cluster{"Samples to Read":i32, "Rate (Hz)":dbl, "Amplitude (mV/pA)":dbl, "Offset (mV/pA)":dbl, "Frequency (Hz)":dbl, "duty cycle (%)":dbl, "phase":dbl}
  T18 = cluster{" Iprot":bool, " Vprot":bool, " Imemtest":bool, " Vmemtest":bool}
  T19 = enum32{"PhaseA", "PhaseB", "PhaseC", "PhaseD", "PhaseE", "PhaseF", "PhaseG", "PhaseH", "PhaseI", "PhaseJ", "PhaseK", "PhaseL", "PhaseM", "PhaseN"}
  T20 = enum32{"Single Jump", "Solution Change", "Voltage Step", "Voltage Ramp", "Voltage Pulse", "Jump Train", "Paired Pulse", "Single Manip Jump", "Gap Free", "Multi M. Jump", "Current Pulse", "Current Ramp", "Gap Free Iclamp"}
  T21 = cluster{"Which Position to use for Experiment":enum16{"Jumper Safe Position", "Experiment Safe Position", "Jumper Position A", "Jumper Position B", "Jumper Position C", "Jumper Position o-A", "Jumper Position A-o", "Jumper Position A-B", "Jumper Position B-A", "Jumper Position B-C", "Jumper Position C-B", "Jumper Position C-o", "Jumper Position o-C", "Don't Move"}, "Start Position (N)":string, "Jump Position (m)":string, "Duration (s)":dbl, "Delay (s)":dbl, "Pulse Width (s)":dbl, "Valve 1 Position":i16, "Valve 2 Position":i16, "Replicates":dbl, "Vholding (mV)":dbl, "Valve 3 Position":i16, "valve 1 used now?":bool, "valve 2 used now?":bool, "valve 3 used now? ":bool, "protocol Preview":waveform(dbl)[]}
  T22 = cluster{"Which Position to use for Experiment":enum16{"Jumper Safe Position", "Experiment Safe Position", "Jumper Position A", "Jumper Position B", "Jumper Position C", "Jumper Position o-A", "Jumper Position A-o", "Jumper Position A-B", "Jumper Position B-A", "Jumper Position B-C", "Jumper Position C-B", "Jumper Position C-o", "Jumper Position o-C", "Don't Move"}, "Duration (s)":dbl, "Delay (s)":dbl, "Pulse Width (s)":dbl, "Which Valve to Change?":i16, "Valve Jump Position":i16, "Replicates":dbl, "Vholding (mV)":dbl, "valve 1 used now?":bool, "valve 2 used now?":bool, "valve 3 used now? ":bool, "Valve 1 Position":i16, "Valve 2 Position":i16, "Valve 3 Position":i16, "protocol Preview":waveform(dbl)[]}
  T23 = cluster{"Which Position to use for Experiment":enum16{"Jumper Safe Position", "Experiment Safe Position", "Jumper Position A", "Jumper Position B", "Jumper Position C", "Jumper Position o-A", "Jumper Position A-o", "Jumper Position A-B", "Jumper Position B-A", "Jumper Position B-C", "Jumper Position C-B", "Jumper Position C-o", "Jumper Position o-C", "Don't Move"}, "Duration (s)":dbl, "Delay (s)":dbl, "Step Width (s)":dbl, "Voltage Start (mV)":dbl, "Voltage Step (mV)":dbl, "Replicates":dbl, "Voltage End (mV)":dbl, "Number of Step":dbl, "Vholding (mV)":dbl, "Valve 1 Position":i16, "Valve 2 Position":i16, "Valve 3 Position":i16, "valve 1 used now?":bool, "valve 2 used now?":bool, "valve 3 used now? ":bool, "Total Step Time (s)":dbl, "Maintain Final Voltage until end?":bool, "protocol Preview":waveform(dbl)[]}